vi "Velociprobe_Nanopositioner_Control_RT.vi"() -> ()   [LabVIEW 2015] (continued)
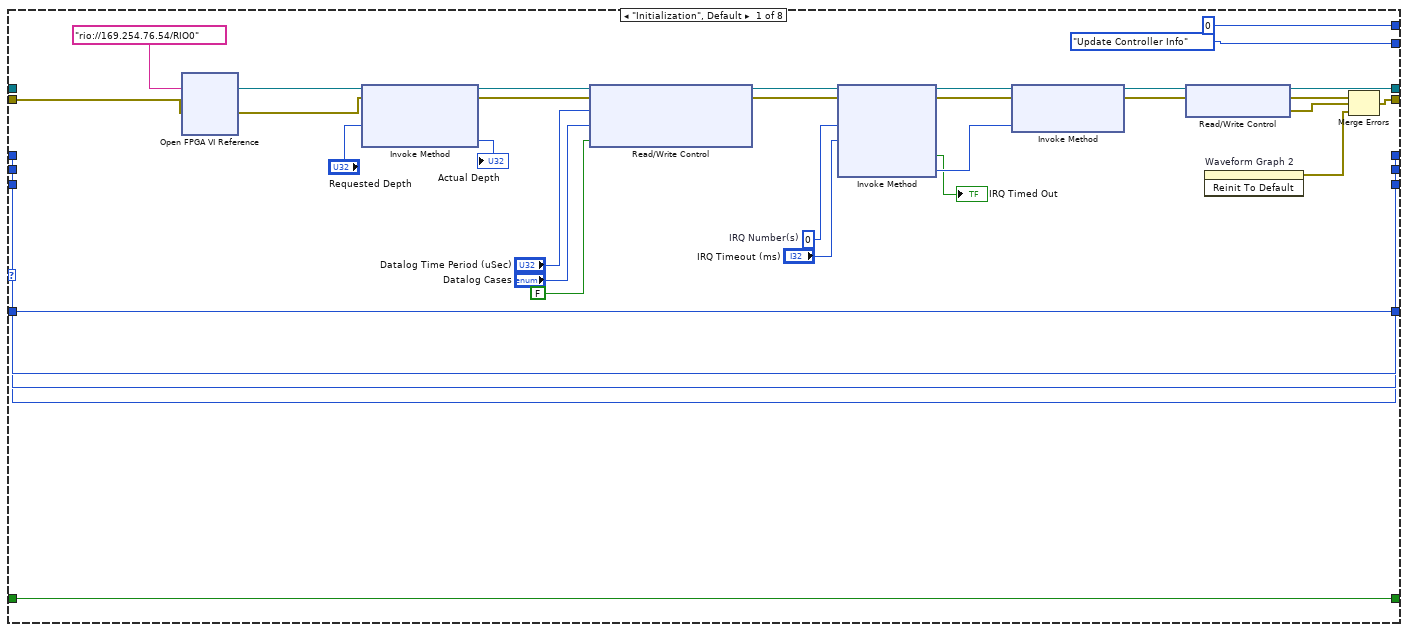
[diagram p2: hidden frame]
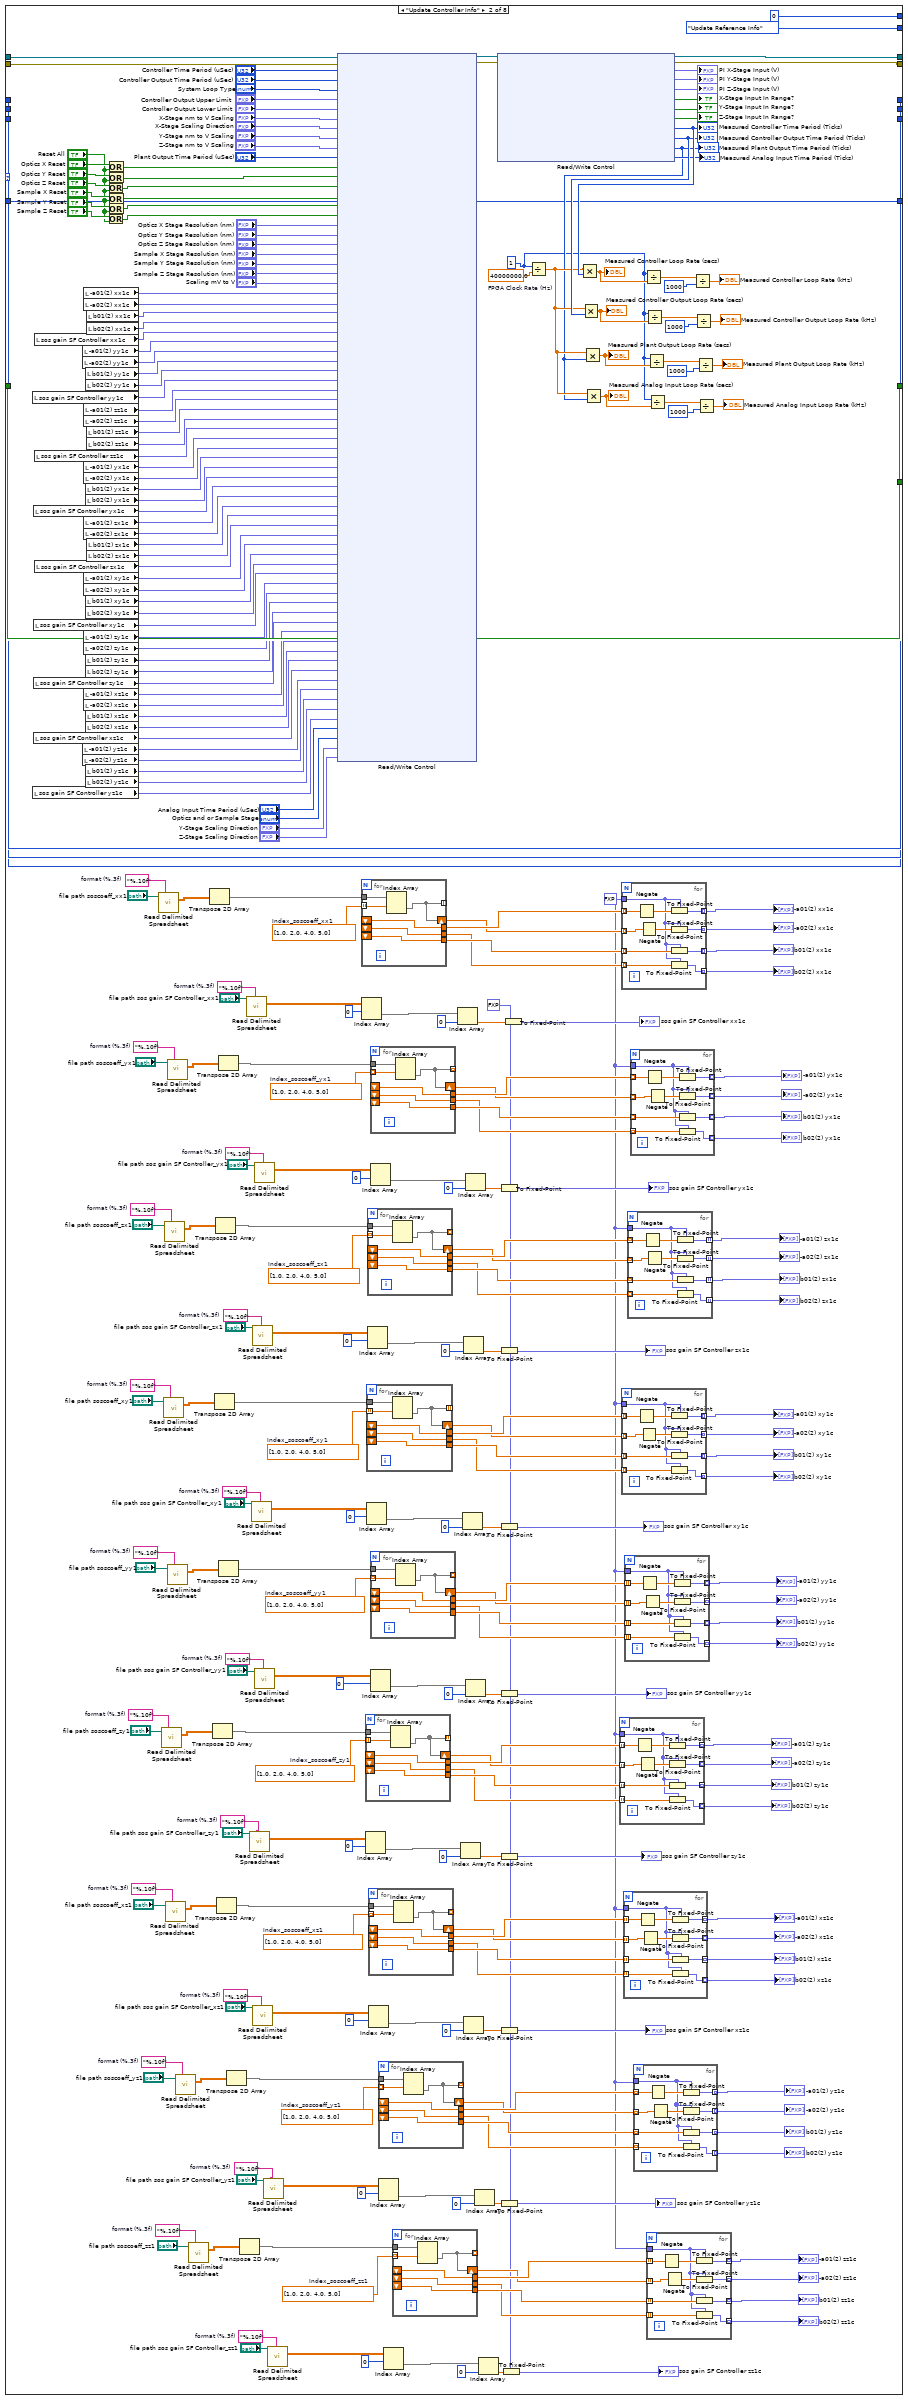
[diagram p3: hidden frame]
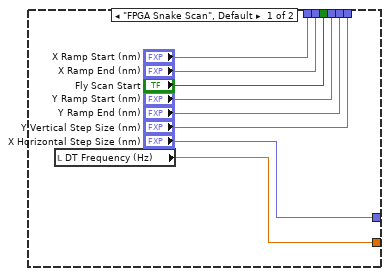
[diagram p4: hidden frame]
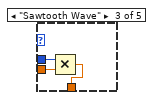
[diagram p6: hidden frame]
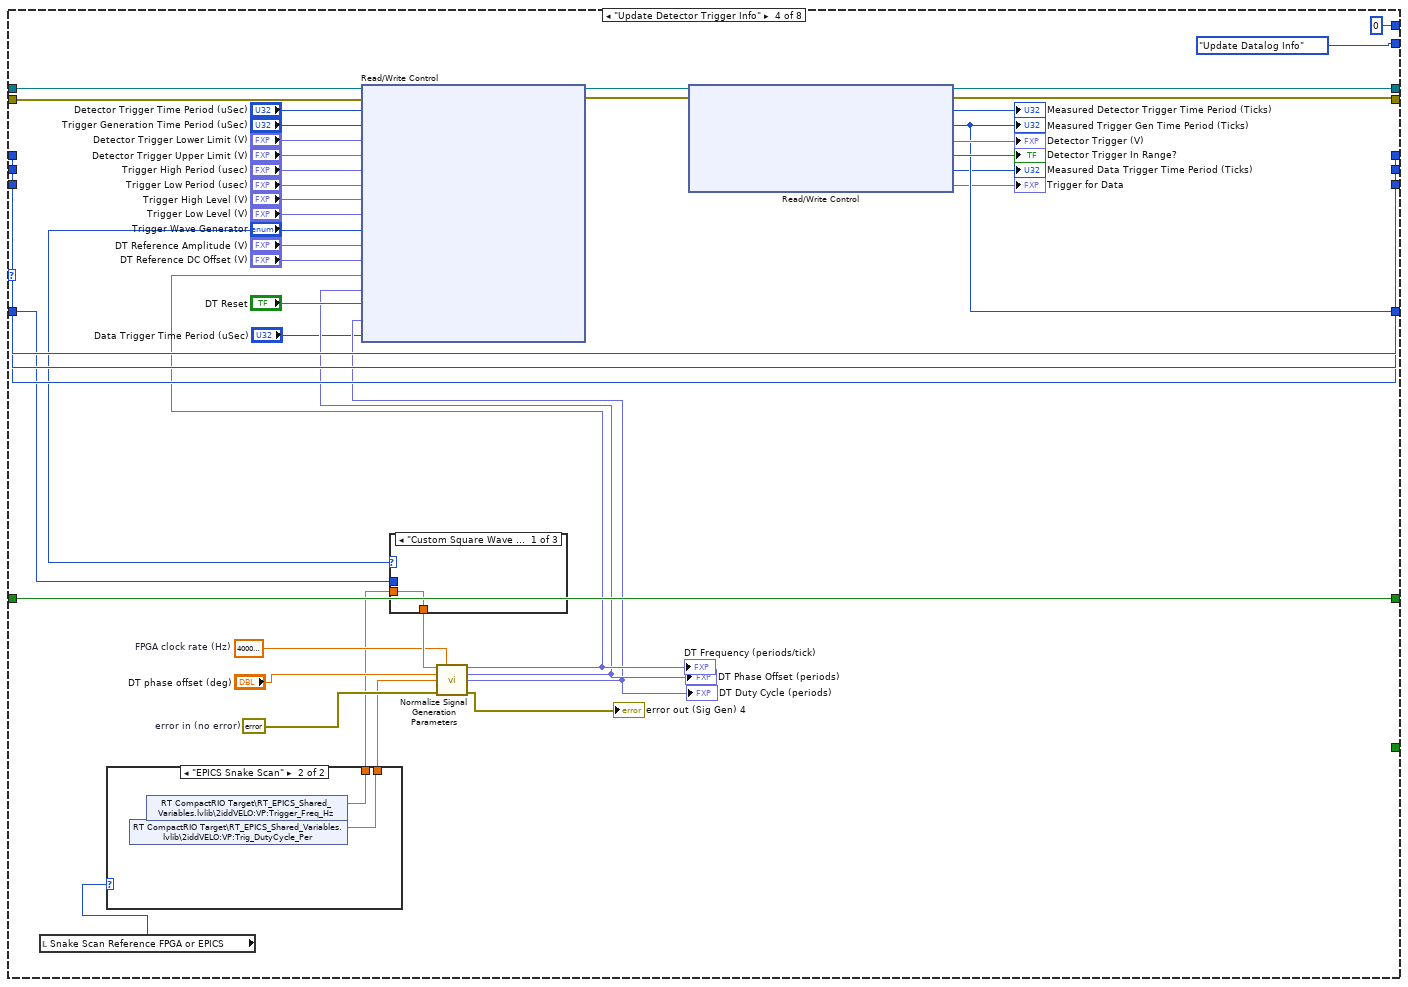
[diagram p15: hidden frame]
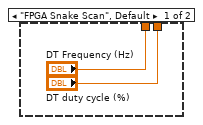
[diagram p16: hidden frame]
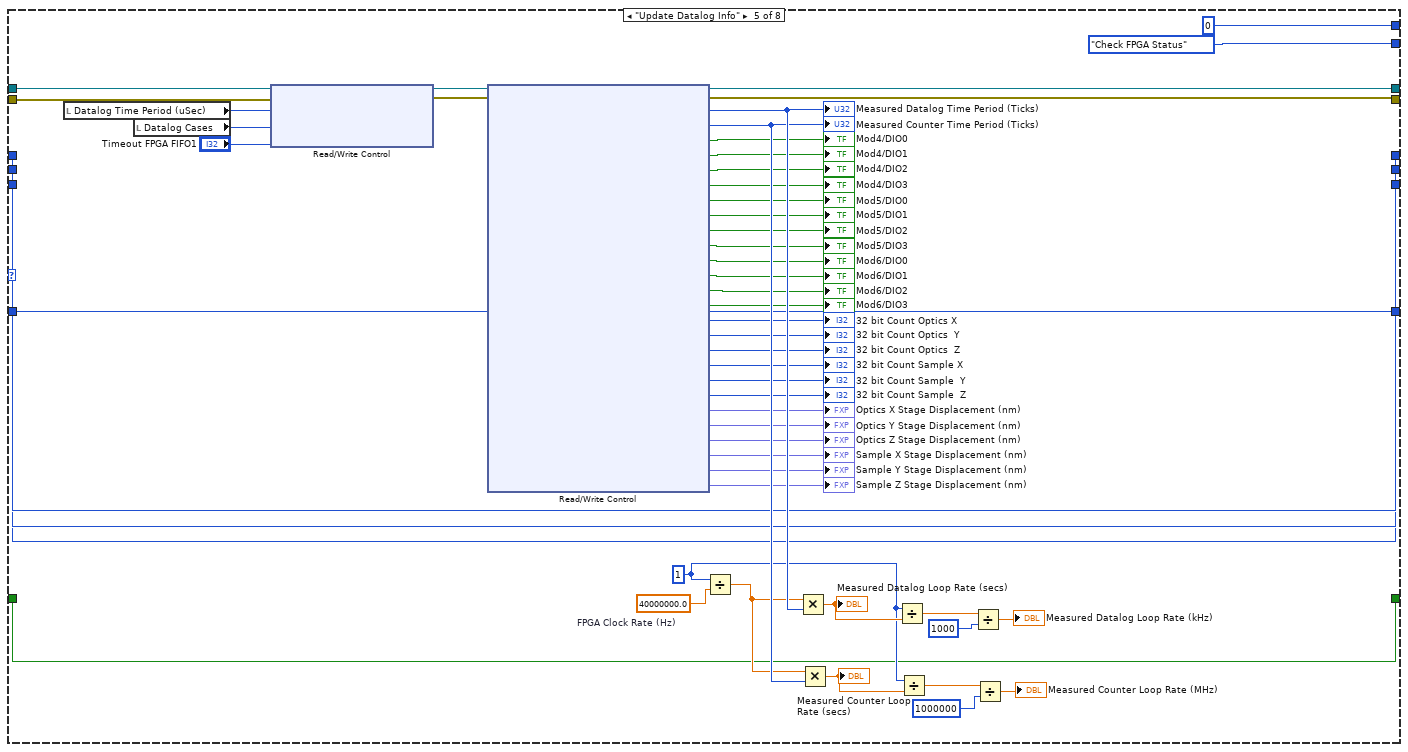
[diagram p19: hidden frame]
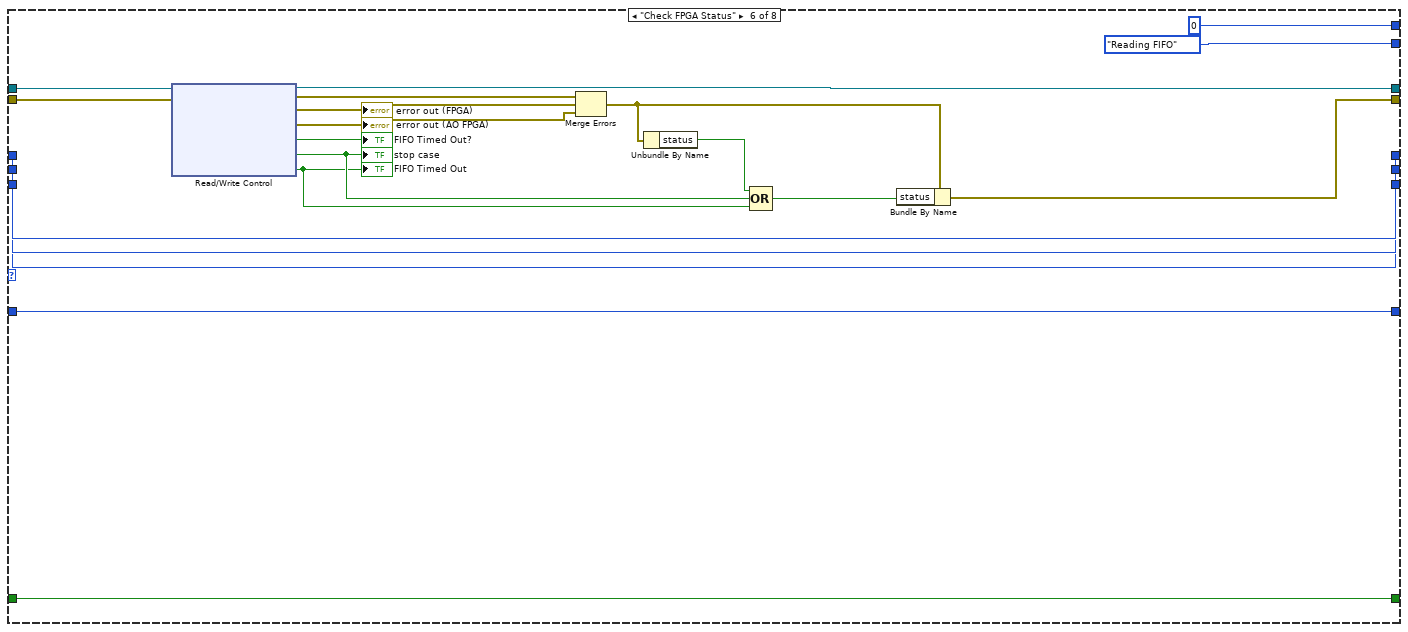
[diagram p20: hidden frame]
          tunnel: w287 -> [w491] mode=indexing
          tunnel: [w490] -> w291 mode=indexing
          tunnel: [w489] -> w290 mode=indexing
          tunnel: [w488] -> w289 mode=indexing
          tunnel: w104 -> [w485]
          n205 = Negate(x=w495) -> (-x=w487:dbl)
          n206 = Negate(x=w493) -> (-x=w486:dbl)
          n207 = To Fixed-Point(fixed-point type=w485, number=w487) -> (fixed-point=w494:fxp<+/-,64,9>)
          n208 = To Fixed-Point(fixed-point type=w485, number=w486) -> (fixed-point=w490:fxp<+/-,64,9>)
          n209 = To Fixed-Point(fixed-point type=w485, number=w492) -> (fixed-point=w489:fxp<+/-,64,9>)
          n210 = To Fixed-Point(fixed-point type=w485, number=w491) -> (fixed-point=w488:fxp<+/-,64,9>)
        }
        "-a01(2) zz1c" <- w292
        "-a02(2) zz1c" <- w291
        "b01(2) zz1c" <- w290
        "b02(2) zz1c" <- w289
        n211 = Divide(x=w81, y=w87) -> (x/y=w86:dbl)
        n212 = Divide(x=w362, y=1000) -> (x/y=→"Measured Controller Loop Rate (kHz)":dbl)
        n213 = Divide(x=w358, y=1000) -> (x/y=→"Measured Controller Output Loop Rate (kHz)":dbl)
        n214 = Divide(x=w354, y=1000) -> (x/y=→"Measured Plant Output Loop Rate (kHz)":dbl)
        n215 = Divide(x=w86, y=1000) -> (x/y=→"Measured Analog Input Loop Rate (kHz)":dbl)
      }
      frame "Update Reference Info" {
        w607 = 40000000.0  # FPGA Clock Rate (Hz)
        w601 = 1
        w614 = 40000000.0  # FPGA Clock Rate (Hz)
        w608 = 1
        w619 = errorcluster {"status"=FALSE, "code"=0, "source"=""}  # error in (no error)
        w622 = errorcluster {"status"=FALSE, "code"=0, "source"=""}  # error in (no error)
        w636 = 40000000.0  # FPGA Clock Rate (Hz)
        w630 = 1
        w648 = errorcluster {"status"=FALSE, "code"=0, "source"=""}  # error in (no error)
        w615 = 40000000.0  # FPGA clock rate (Hz)
        n216 = case shown="\"EPICS Snake Scan\"" "Snake Scan Reference FPGA or EPICS" {
          tunnel: ["X Ramp Start (nm)" w668] -> w543
          tunnel: ["X Ramp End (nm)" w667] -> w542
          tunnel: ["Fly Scan Start" w666] -> w541
          tunnel: ["Y Ramp Start (nm)" w665] -> w540
          tunnel: ["Y Ramp End (nm)" w664] -> w539
          tunnel: ["Y Vertical Step Size (nm)" w663] -> w538
          tunnel: ["X Horizontal Step Size (nm)" w662] -> w537
          tunnel: [w652 w660] -> w536
          frame "FPGA Snake Scan", Default {
            n217 = local read "DT Frequency (Hz)"() -> (w652:dbl)
          }
          frame "EPICS Snake Scan" {
            w661 = fxp<+/-,16,16> 0.0 ("fixed-point type")
            n218 = shared-variable "RT CompactRIO Target\\RT_EPICS_Shared_Variables.lvlib\\2iddVELO:VP:Trigger_Freq_Hz"() -> (w660:dbl)  [unwired: 1 in, 1 out]
            n219 = shared-variable "RT CompactRIO Target\\RT_EPICS_Shared_Variables.lvlib\\2iddVELO:VP:Y_Step_Size_nm"() -> (w670:dbl)  [unwired: 1 in, 1 out]
            n220 = shared-variable "RT CompactRIO Target\\RT_EPICS_Shared_Variables.lvlib\\2iddVELO:VP:X_Step_Size_nm"() -> (w669:dbl)  [unwired: 1 in, 1 out]
            n221 = shared-variable "RT CompactRIO Target\\RT_EPICS_Shared_Variables.lvlib\\2iddVELO:VP:Flyscan_Start"() -> (w666:bool)  [unwired: 1 in, 1 out]
            n222 = shared-variable "RT CompactRIO Target\\RT_EPICS_Shared_Variables.lvlib\\2iddVELO:VP:X_Start_nm"() -> (w674:dbl)  [unwired: 1 in, 1 out]
            n223 = shared-variable "RT CompactRIO Target\\RT_EPICS_Shared_Variables.lvlib\\2iddVELO:VP:Y_Start_nm"() -> (w672:dbl)  [unwired: 1 in, 1 out]
            n224 = shared-variable "RT CompactRIO Target\\RT_EPICS_Shared_Variables.lvlib\\2iddVELO:VP:X_End_nm"() -> (w673:dbl)  [unwired: 1 in, 1 out]
            n225 = shared-variable "RT CompactRIO Target\\RT_EPICS_Shared_Variables.lvlib\\2iddVELO:VP:Y_End_nm"() -> (w671:dbl)  [unwired: 1 in, 1 out]
            n226 = To Fixed-Point(fixed-point type=w661, number=w674) -> (fixed-point=w668:fxp<+/-,16,16>)
            n227 = To Fixed-Point(fixed-point type=w661, number=w673) -> (fixed-point=w667:fxp<+/-,16,16>)
            n228 = To Fixed-Point(fixed-point type=w661, number=w672) -> (fixed-point=w665:fxp<+/-,16,16>)
            n229 = To Fixed-Point(fixed-point type=w661, number=w671) -> (fixed-point=w664:fxp<+/-,16,16>)
            n230 = To Fixed-Point(fixed-point type=w661, number=w670) -> (fixed-point=w663:fxp<+/-,16,16>)
            n231 = To Fixed-Point(fixed-point type=w661, number=w669) -> (fixed-point=w662:fxp<+/-,16,16>)
          }
        }
        n232 = local read "X Ramp Period (usec)"() -> (w550:fxp<+,24,24>)
        n233 = local read "Y Ramp Period (usec)"() -> (w551:fxp<+,24,24>)
        n234 = case shown="\"Constant\", Default" "Z Reference Wave Selection" {
          tunnel: "Z frequency (Hz)" -> [w675 w676 w678 w680 w681]
          tunnel: [w675 w676 w677 w680 w681] -> w576
          tunnel: w575 -> [_ _ w679 _ _]
          frame "Constant", Default {
          }
          frame "Sine Wave" {
          }
          frame "Sawtooth Wave" {
            n235 = Multiply(x=w679, y=w678) -> (x*y=w677:dbl)
          }
          frame "Square Wave" {
          }
          frame "Filtered White Noise" {
          }
        }
        n236 = case shown="\"Constant\", Default" "Y Reference Wave Selection" {
          tunnel: "Y frequency (Hz)" -> [w682 w683 w684 w685]
          tunnel: [w682 w683 w684 w685] -> w581
          tunnel: w578 -> [_ _ _ _]
          frame "Constant", Default {
          }
          frame "Sine Wave" {
          }
          frame "Custom Ramp Wave" {
          }
          frame "Filtered White Noise" {
          }
        }
        n237 = case shown="\"Custom Up Down Ramp\"" "X Reference Wave Selection" {
          tunnel: "X frequency (Hz)" -> [w686 w687 w688 w689]
          tunnel: [w686 w687 w688 w689] -> w585
          tunnel: w583 -> [_ _ _ _]
          frame "Constant", Default {
          }
          frame "Sine Wave" {
          }
          frame "Custom Up Down Ramp" {
          }
          frame "Filtered White Noise" {
          }
        }
        n238 = call <vilib>:"Normalize Signal Generation Parameters.vi"("frequency (Hz)"=w581, "FPGA clock rate (Hz)"=w615, "phase offset (deg)"="Y phase offset (deg)", "error in (no error)"=w622) -> ("frequency (periods/tick)"=w618:fxp<+,32,0>, "phase offset (periods)"=w617:fxp<+,32,0>, "error out"=→"error out (Sig Gen) 2":errorcluster)  [unwired: 6 in, 3 out]
        "Y frequency (periods/tick)" <- w618
        "Y phase offset (periods)" <- w617
        n239 = call <vilib>:"Normalize Signal Generation Parameters.vi"("frequency (Hz)"=w576, "FPGA clock rate (Hz)"=w615, "phase offset (deg)"="Z phase offset (deg)", "error in (no error)"=w619) -> ("frequency (periods/tick)"=w616:fxp<+,32,0>, "phase offset (periods)"=w594:fxp<+,32,0>, "error out"=→"error out (Sig Gen) 3":errorcluster)  [unwired: 6 in, 3 out]
        "Z frequency (periods/tick)" <- w616
        "Z phase offset (periods)" <- w594
        n240 = call <vilib>:"Normalize Signal Generation Parameters.vi"("frequency (Hz)"=w585, "FPGA clock rate (Hz)"=w615, "phase offset (deg)"="X phase offset (deg)", "error in (no error)"=w648) -> ("frequency (periods/tick)"=w647:fxp<+,32,0>, "phase offset (periods)"=w625:fxp<+,32,0>, "error out"=→"error out (Sig Gen)":errorcluster)  [unwired: 6 in, 3 out]
        "X frequency (periods/tick)" <- w647
        "X phase offset (periods)" <- w625
        n241 = xnode "Read/Write Control"("FPGA VI Reference In"=w535, "error in"=w534, "X Reference Time Period (uSec)"="X Reference Time Period (uSec)", "Y Reference Time Period (uSec)"="Y Reference Time Period (uSec)", "Z Reference Time Period (uSec)"="Z Reference Time Period (uSec)", "X Reference Wave Selection"="X Reference Wave Selection", "Y Reference Wave Selection"="Y Reference Wave Selection", "Z Reference Wave Selection"="Z Reference Wave Selection", "X Reference Reset"="X Reference Reset", "Y Reference Reset"="Y Reference Reset", "Z Reference Reset"="Z Reference Reset", "X Reference Amplitude (nm)"="X Reference Amplitude (nm)", "Y Reference Amplitude (nm)"="Y Reference Amplitude (nm)", "Z Reference Amplitude (nm)"="Z Reference Amplitude (nm)", "X Frequency (periods/tick)"=w647, "X Phase Offset (periods)"=w625, "Y Frequency (periods/tick)"=w618, "Y Phase Offset (periods)"=w617, "Z Frequency (periods/tick)"=w616, "Z Phase Offset (periods)"=w594, "X Reference DC Offset (nm)"="X Reference DC Offset (nm)", "Y Reference DC Offset (nm)"="Y Reference DC Offset (nm)", "Z Reference DC Offset (nm)"="Z Reference DC Offset (nm)", "X White Noise Amplitude"="X White Noise Amplitude", "X White Noise Seed"="X White Noise Seed", "Y White Noise Amplitude"="Y White Noise Amplitude", "Y White Noise Seed"="Y White Noise Seed", "Z White Noise Amplitude"="Z White Noise Amplitude", "Z White Noise Seed"="Z White Noise Seed", "Mod 3 AI0 V to nm Scaling"="Mod 3 AI0 V to nm Scaling", "Mod 3 AI1 V to nm Scaling"="Mod 3 AI1 V to nm Scaling", "Mod 3 AI2 V to nm Scaling"="Mod 3 AI2 V to nm Scaling", "X Ramp Period (usec)"=w550, "X Ramp Start (nm)"=w543, "X Ramp End (nm)"=w542, "X Start Marker (nm)"="X Start Marker (nm)", "Fly Scan Start"=w541, "Y Ramp Period (usec)"=w551, "Y Ramp Start (nm)"=w540, "Y Ramp End (nm)"=w539, "Y Ramp Drop Size (nm)"=w538, "Y Start Marker (nm)"="Y Start Marker (nm)") -> ("FPGA VI Reference Out"=w533:refnum<k20>, "error out"=w532:errorcluster)
        n242 = local read "Y Ramp Start (nm)"() -> (w549:fxp<+/-,16,16>)
        n243 = local read "X Ramp Start (nm)"() -> (w547:fxp<+/-,16,16>)
        n244 = local read "Y Ramp End (nm)"() -> (w548:fxp<+/-,16,16>)
        n245 = local read "X Ramp End (nm)"() -> (w546:fxp<+/-,16,16>)
        n246 = xnode "Read/Write Control"("FPGA VI Reference In"=w533, "error in"=w532) -> ("FPGA VI Reference Out"=w530:refnum<k20>, "error out"=w531:errorcluster, "X Stage Reference (nm)"=→"X Stage Reference (nm)":fxp<+/-,58,25>, "Y Stage Reference (nm)"=→"Y Stage Reference (nm)":fxp<+/-,58,25>, "Z Stage Reference (nm)"=→"Z Stage Reference (nm)":fxp<+/-,58,25>, "Measured X Reference Time Period (Ticks)"=w584:u32, "Measured Y Reference Time Period (Ticks)"=w580:u32, "Measured Z Reference Time Period (Ticks)"=w579:u32, "Fly Scan Running"=→"Fly Scan Running":bool, "Continue Run"=→"Continue Run":bool)
        "Measured X Reference Time Period (Ticks)" <- w584
        "Measured Y Reference Time Period (Ticks)" <- w580
        "Measured Z Reference Time Period (Ticks)" <- w579
        n247 = Subtract(x=w549, y=w548) -> (x-y=w567:fxp<+/-,17,17>)
        n248 = Subtract(x=w547, y=w546) -> (x-y=w565:fxp<+/-,17,17>)
        n249 = Absolute Value(x=w567) -> (abs(x)=w558:fxp<+,16,16>)
        n250 = Absolute Value(x=w565) -> (abs(x)=w564:fxp<+,16,16>)
        n251 = local read "Y Vertical Step Size (nm)"() -> (w545:fxp<+/-,16,16>)
        n252 = Divide(x=w564, y=w537) -> (x/y=w562:fxp<+/-,33,17>)
        "# of Points per Line" <- w562
        n253 = Divide(x=w630, y=w636) -> (x/y=w631:dbl)
        n254 = Divide(x=w608, y=w614) -> (x/y=w609:dbl)
        n255 = Divide(x=w601, y=w607) -> (x/y=w602:dbl)
        n256 = Divide(x=w562, y=w536) -> (x/y=w554:dbl)
        "sec per line" <- w554
        n257 = Multiply(x=w631, y=w584) -> (x*y=w635:dbl)
        "Measured X Reference Loop Rate (secs)" <- w635
        n258 = Multiply(x=w609, y=w580) -> (x*y=w613:dbl)
        "Measured Y Reference Loop Rate (secs)" <- w613
        n259 = Divide(x=w558, y=w545) -> (x/y=w559:fxp<+/-,33,17>)
        n260 = Multiply(x=w602, y=w579) -> (x*y=w606:dbl)
        "Measured Z Reference Loop Rate (secs)" <- w606
        n261 = Add(x=w559, y=fxp<+,16,16> 1.0) -> (x+y=w553:fxp<+/-,34,18>)
        "# of Hor Lines" <- w553
        n262 = Multiply(x=w554, y=1000000.0) -> (x*y=w557:dbl)
        "X Ramp Period DBL (usec)" <- w557
        n263 = Reciprocal(x=w554) -> (1/x=→"line per sec (Hz)":dbl)
        n264 = Divide(x=w630, y=w635) -> (x/y=w634:dbl)
        n265 = Divide(x=w608, y=w613) -> (x/y=w612:dbl)
        n266 = To Fixed-Point(fixed-point type=fxp<+,24,24> 0.0, number=w557) -> (fixed-point=→"X Ramp Period (usec)" →"Y Ramp Period (usec)":fxp<+,24,24>)
        n267 = Multiply(x=w554, y=w553) -> (x*y=→"Total Scan Time (sec)":dbl)
        n268 = Divide(x=w601, y=w606) -> (x/y=w605:dbl)
        n269 = Multiply(x=w553, y=w562) -> (x*y=→"# Total Trigger Points":fxp<+/-,64,34>)
        n270 = Divide(x=w634, y=1000) -> (x/y=→"Measured X Reference Loop Rate (kHz)":dbl)
        n271 = Divide(x=w612, y=1000) -> (x/y=→"Measured Y Reference Loop Rate (kHz)":dbl)
        n272 = Divide(x=w605, y=1000) -> (x/y=→"Measured Z Reference Loop Rate (kHz)":dbl)
      }
      frame "Update Detector Trigger Info" {
        w708 = 40000000.0  # FPGA clock rate (Hz)
        w710 = errorcluster {"status"=FALSE, "code"=0, "source"=""}  # error in (no error)
        n273 = local read "Snake Scan Reference FPGA or EPICS"() -> (w701:enum16{"FPGA Snake Scan", "EPICS Snake Scan"})
        n274 = case shown="\"EPICS Snake Scan\"" w701 {
          tunnel: ["DT Frequency (Hz)" w736] -> w700
          tunnel: ["DT duty cycle (%)" w735] -> w699
          frame "FPGA Snake Scan", Default {
          }
          frame "EPICS Snake Scan" {
            n275 = shared-variable "RT CompactRIO Target\\RT_EPICS_Shared_Variables.lvlib\\2iddVELO:VP:Trig_DutyCycle_Per"() -> (w735:dbl)  [unwired: 1 in, 1 out]
            n276 = shared-variable "RT CompactRIO Target\\RT_EPICS_Shared_Variables.lvlib\\2iddVELO:VP:Trigger_Freq_Hz"() -> (w736:dbl)  [unwired: 1 in, 1 out]
          }
        }
        n277 = case shown="\"Custom Square Wave \", Default" "Trigger Wave Generator" {
          tunnel: w700 -> [w737 w738 w739]
          tunnel: [w737 w738 w739] -> w709
          tunnel: w702 -> [_ _ _]
          frame "Custom Square Wave ", Default {
          }
          frame "Square Wave 1" {
          }
          frame "Square Wave 2" {
          }
        }
        n278 = call <vilib>:"Normalize Signal Generation Parameters.vi"("frequency (Hz)"=w709, "FPGA clock rate (Hz)"=w708, "phase offset (deg)"="DT phase offset (deg)", "duty cycle (%)"=w699, "error in (no error)"=w710) -> ("frequency (periods/tick)"=w706:fxp<+,32,0>, "phase offset (periods)"=w705:fxp<+,32,0>, "duty cycle (periods)"=w704:fxp<+,32,0>, "error out"=→"error out (Sig Gen) 4":errorcluster)  [unwired: 5 in, 2 out]
        "DT Frequency (periods/tick)" <- w706
        "DT Phase Offset (periods)" <- w705
        "DT Duty Cycle (periods)" <- w704
        n279 = xnode "Read/Write Control"("FPGA VI Reference In"=w698, "error in"=w697, "Detector Trigger Time Period (uSec)"="Detector Trigger Time Period (uSec)", "Trigger Generation Time Period (uSec)"="Trigger Generation Time Period (uSec)", "Detector Trigger Lower Limit (V)"="Detector Trigger Lower Limit (V)", "Detector Trigger Upper Limit (V)"="Detector Trigger Upper Limit (V)", "Trigger High Period (usec)"="Trigger High Period (usec)", "Trigger Low Period (usec)"="Trigger Low Period (usec)", "Trigger High Level (V)"="Trigger High Level (V)", "Trigger Low Level (V)"="Trigger Low Level (V)", "Trigger Wave Generator"="Trigger Wave Generator", "DT Reference Amplitude (V)"="DT Reference Amplitude (V)", "DT Reference DC Offset (V)"="DT Reference DC Offset (V)", "DT Frequency (periods/tick)"=w706, "DT Phase Offset (periods)"=w705, "DT Reset"="DT Reset", "DT Duty Cycle (periods)"=w704, "Data Trigger Time Period (uSec)"="Data Trigger Time Period (uSec)") -> ("FPGA VI Reference Out"=w696:refnum<k20>, "error out"=w695:errorcluster)
        n280 = xnode "Read/Write Control"("FPGA VI Reference In"=w696, "error in"=w695) -> ("FPGA VI Reference Out"=w694:refnum<k20>, "error out"=w693:errorcluster, "Measured Detector Trigger Time Period (Ticks)"=→"Measured Detector Trigger Time Period (Ticks)":u32, "Measured Trigger Gen Time Period (Ticks)"=w703:u32, "Detector Trigger (V)"=→"Detector Trigger (V)":fxp<+/-,20,5>, "Detector Trigger In Range?"=→"Detector Trigger In Range?":bool, "Measured Data Trigger Time Period (Ticks)"=→"Measured Data Trigger Time Period (Ticks)":u32, "Trigger for Data"=→"Trigger for Data":fxp<+/-,58,25>)
        "Measured Trigger Gen Time Period (Ticks)" <- w703
      }
      frame "Update Datalog Info" {
        w784 = 40000000.0  # FPGA Clock Rate (Hz)
        w773 = 1
        n281 = local read "Datalog Time Period (uSec)"() -> (w771:u32)
        n282 = local read "Datalog Cases"() -> (w770:T6)
        n283 = xnode "Read/Write Control"("FPGA VI Reference In"=w745, "error in"=w744, "Datalog Time Period (uSec)"=w771, "Datalog Cases"=w770, "Timeout FPGA FIFO1"="Timeout FPGA FIFO1") -> ("FPGA VI Reference Out"=w743:refnum<k20>, "error out"=w742:errorcluster)
        n284 = xnode "Read/Write Control"("FPGA VI Reference In"=w743, "error in"=w742) -> ("FPGA VI Reference Out"=w740:refnum<k20>, "error out"=w741:errorcluster, "Measured Datalog Time Period (Ticks)"=w783:u32, "Measured Counter Time Period (Ticks)"=w781:u32, "Mod4/DIO0"=→"Mod4/DIO0":bool, "Mod4/DIO1"=→"Mod4/DIO1":bool, "Mod4/DIO2"=→"Mod4/DIO2":bool, "Mod4/DIO3"=→"Mod4/DIO3":bool, "Mod5/DIO0"=→"Mod5/DIO0":bool, "Mod5/DIO1"=→"Mod5/DIO1":bool, "Mod5/DIO2"=→"Mod5/DIO2":bool, "Mod5/DIO3"=→"Mod5/DIO3":bool, "Mod6/DIO0"=→"Mod6/DIO0":bool, "Mod6/DIO1"=→"Mod6/DIO1":bool, "Mod6/DIO2"=→"Mod6/DIO2":bool, "Mod6/DIO3"=→"Mod6/DIO3":bool, "32 bit Count Optics X"=→"32 bit Count Optics X":i32, "32 bit Count Optics  Y"=→"32 bit Count Optics  Y":i32, "32 bit Count Optics  Z"=→"32 bit Count Optics  Z":i32, "32 bit Count Sample X"=→"32 bit Count Sample X":i32, "32 bit Count Sample  Y"=→"32 bit Count Sample  Y":i32, "32 bit Count Sample  Z"=→"32 bit Count Sample  Z":i32, "Optics X Stage Displacement (nm)"=→"Optics X Stage Displacement (nm)":fxp<+/-,58,25>, "Optics Y Stage Displacement (nm)"=→"Optics Y Stage Displacement (nm)":fxp<+/-,58,25>, "Optics Z Stage Displacement (nm)"=→"Optics Z Stage Displacement (nm)":fxp<+/-,58,25>, "Sample X Stage Displacement (nm)"=→"Sample X Stage Displacement (nm)":fxp<+/-,58,25>, "Sample Y Stage Displacement (nm)"=→"Sample Y Stage Displacement (nm)":fxp<+/-,58,25>, "Sample Z Stage Displacement (nm)"=→"Sample Z Stage Displacement (nm)":fxp<+/-,58,25>)
        "Measured Datalog Time Period (Ticks)" <- w783
        "Measured Counter Time Period (Ticks)" <- w781
        n285 = Divide(x=w773, y=w784) -> (x/y=w780:dbl)
        n286 = Multiply(x=w780, y=w783) -> (x*y=w791:dbl)
        "Measured Datalog Loop Rate (secs)" <- w791
        n287 = Multiply(x=w780, y=w781) -> (x*y=w787:dbl)
        "Measured Counter Loop Rate (secs)" <- w787
        n288 = Divide(x=w773, y=w791) -> (x/y=w790:dbl)
        n289 = Divide(x=w773, y=w787) -> (x/y=w786:dbl)
        n290 = Divide(x=w790, y=1000) -> (x/y=→"Measured Datalog Loop Rate (kHz)":dbl)
        n291 = Divide(x=w786, y=1000000) -> (x/y=→"Measured Counter Loop Rate (MHz)":dbl)
      }
      frame "Check FPGA Status" {
        n292 = xnode "Read/Write Control"("FPGA VI Reference In"=w797, "error in"=w796) -> ("FPGA VI Reference Out"=w795:refnum<k20>, "error out"=w794:errorcluster, "error out (FPGA)"=w810:errorcluster, "error out (AO FPGA)"=w809:errorcluster, "FIFO Timed Out?"=→"FIFO Timed Out?":bool, "stop case"=w804:bool, "FIFO Timed Out"=w803:bool)
        "error out (FPGA)" <- w810
        "error out (AO FPGA)" <- w809
        "stop case" <- w804
        "FIFO Timed Out" <- w803
        n293 = Merge Errors "Merge Errors"(w794, w810, w809) -> (w805:errorcluster)
        n294 = Unbundle By Name "Unbundle By Name"(w805) -> ("status"=w808:bool)
        n295 = Compound Arithmetic op=OR(w808, w804, w803) -> (w806:bool)
        n296 = Bundle By Name "Bundle By Name"(cluster=w805, "status"=w806) -> (w793:errorcluster)
      }
      frame "Reading FIFO" {
        w863 = 0.0  # t0
        n297 = xnode "Read/Write Control"("FPGA VI Reference In"=w820, "error in"=w819) -> ("FPGA VI Reference Out"=w818:refnum<k20>, "error out"=w817:errorcluster, "Number of Data Strings"=→"Number of Data Strings":i32)
        n298 = Greater?(x="Write Data", y=w848) -> (0:w845:bool)
        n299 = case shown="True" w845 {
          tunnel: w819 -> [w879 w882]
          tunnel: [w879 w883] -> w843
          frame False {
          }
          frame True {
            n300 = call "Data_Write.vi"("Command List"=Data_Write_Control."Initialize", "name"="name", "error initialize"=w882) -> ("error out"=w883:errorcluster)  [unwired: 6 in]
          }
        }
        n301 = local read "Datalog Time Period (uSec)"() -> (w861:u32)
        n302 = Less?(x="Write Data", y=w848) -> (x < y?=w844:bool)
        n303 = Multiply(x=1e-06, y=w861) -> (x*y=w853:dbl)
        "Datalog Time Period (sec)" <- w853
        n304 = Divide(x=1.0, y=w853) -> (x/y=w857:dbl)
        "Datalog Rate (Hz)" <- w857
        n305 = Multiply(x="FIFO Time Period", y=w857) -> (x*y=w855:dbl)
        n306 = Multiply(x=5 ("Number of Data Strings 2"), y=w855) -> (x*y=w854:dbl)
        n307 = To Unsigned Long Integer(number=w854) -> (unsigned 32bit integer=w850:u32)
        "Number of Elements" <- w850
        n308 = xnode "Invoke Method"("FPGA VI Reference In"=w818, "error in"=w817, "Number of Elements"=w850, "Timeout (ms)"="Timeout (ms)") -> ("FPGA VI Reference Out"=w816:refnum<k20>, "error out"=w815:errorcluster, "Data"=w851:fxp<+/-,58,25>[], "Elements Remaining"=→"Elements Remaining" →"Elements Remaining Waveform Chart" →"Elements Remaining Waveform Chart 3":u32)
        "Data" <- w851
        n309 = Decimate 1D Array "Decimate 1D Array"(w851) -> (w834:fxp<+/-,58,25>[], w825:fxp<+/-,58,25>[], w824:fxp<+/-,58,25>[], w823:fxp<+/-,58,25>[], w821:fxp<+/-,58,25>[])
        n310 = Build Array "Build Array"(w834, w825, w824, w823, w821) -> (w864:fxp<+/-,58,25>[][])
        n311 = To Double Precision Float(number=w864) -> (double precision float=w859:dbl[][])
        n312 = Transpose 2D Array(2D array=w859) -> (transposed array=w841:dbl[][])
        n313 = case shown="True" "Write Data" {
          tunnel: w843 -> [w871 w877]
          tunnel: [w871 w878] -> w842
          tunnel: w841 -> [_ w872]
          frame False {
          }
          frame True {
            w875 = "%8f"  # format string
            w874 = ","  # delimiter (Tab)
            n314 = Array To Spreadsheet String(delimiter (Tab)=w874, array=w872, 3:w875) -> (spreadsheet string=w873:string)
            n315 = call "Data_Write.vi"("Command List"=Data_Write_Control."Write", "Data"=w873, "error initialize"=w877) -> ("error out"=w878:errorcluster)  [unwired: 6 in]
          }
        }
        n316 = call "Convert to Dynamic Data"("Array"=w834) -> ("Dynamic Data Type"=w832:dynamicdata)  [unwired: 3 in]
        n317 = call "Convert to Dynamic Data2"("Array"=w825) -> ("Dynamic Data Type"=w826:dynamicdata)  [unwired: 3 in]
        n318 = call "Convert to Dynamic Data3"("Array"=w824) -> ("Dynamic Data Type"=w828:dynamicdata)  [unwired: 3 in]
        n319 = call "Convert to Dynamic Data4"("Array"=w823) -> ("Dynamic Data Type"=w827:dynamicdata)  [unwired: 3 in]
        n320 = call "Convert from Dynamic Data"("Dynamic Data Type"=w832) -> ("Array"=w833:dbl[])  [unwired: 3 in]
        n321 = call "Convert from Dynamic Data2"("Dynamic Data Type"=w826) -> ("Array"=w831:dbl[])  [unwired: 3 in]
        n322 = call "Convert from Dynamic Data3"("Dynamic Data Type"=w828) -> ("Array"=w830:dbl[])  [unwired: 3 in]
        n323 = call "Convert from Dynamic Data4"("Dynamic Data Type"=w827) -> ("Array"=w829:dbl[])  [unwired: 3 in]
        n324 = case shown="True" w844 {
          tunnel: w842 -> [w867 w869]
          tunnel: [w867 w870] -> w852
          frame False {
          }
          frame True {
            n325 = call "Data_Write.vi"("Command List"=Data_Write_Control."Close", "error initialize"=w869) -> ("error out"=w870:errorcluster)  [unwired: 7 in]
          }
        }
        n326 = Bundle("Array"=w833, "Array"=w831) -> (→"XY Graph":cluster{"Array":dbl[], "Array":dbl[]})  [unwired: 1 in]
        n327 = Bundle("Array"=w830, "Array"=w829) -> (→"XY Graph 2":cluster{"Array":dbl[], "Array":dbl[]})  [unwired: 1 in]
        n328 = Bundle("t0"=w863, w853, w859) -> (→"Waveform Graph 2":cluster{"t0":dbl, dbl, dbl[][]})  [unwired: 1 in]
        n329 = Merge Errors "Merge Errors"(w815, w852) -> (w814:errorcluster)
      }
      frame "Exit" {
        w896 = TRUE ("Stop")
        n330 = xnode "Invoke Method"("FPGA VI Reference In"=w890, "error in"=w889) -> ("FPGA VI Reference Out"=w888:refnum<k20>, "error out"=w887:errorcluster)
        n331 = xnode "Read/Write Control"("FPGA VI Reference In"=w888, "error in"=w887, "stop case"=TRUE) -> ("FPGA VI Reference Out"=w886:refnum<k20>, "error out"=w885:errorcluster)
        n332 = local write "Stop"(w896) -> ()
        n333 = xnode "Close FPGA VI Reference"("FPGA VI Reference In"=w886, "error in"=w885) -> ("error out"=w884:errorcluster)
      }
    }
    n334 = call "State Control.vi"("Error Input"=w14, "Input States"=w25, "Stop"="Stop") -> ("Output State"=w24:T7)  [unwired: 8 in]
    n335 = node-c288(w31) -> ()  [unwired: 1 out]
  }
  n336 = node-c288(w7) -> (→"Error (RT)":errorcluster, →"Iteration Duration RT Timed-Loop":i64)
  n337 = call <vilib>:"Simple Error Handler.vi"("error in (no error)"=w1) -> ("message"=→"message":string)  [unwired: 4 in, 4 out]
